vi "SMain.vi"() -> ()   [LabVIEW 2011] (continued)
                              tunnel: w1059 -> [_ w1085]
                              tunnel: w1058 -> [_ w1084]
                              tunnel: [TRUE ("Total Reult") w1083] -> w1057
                              tunnel: [_ w1082] -> w1056
                              tunnel: w1055 -> [_ w1081]
                              tunnel: w1054 -> [_ w1080]
                              tunnel: w1053 -> [_ w1079]
                              tunnel: w1052 -> [_ w1078]
                              tunnel: w1050 -> [_ w1077]
                              tunnel: [string[] [] ("NEXT Pair Name") w1076] -> w1047
                              tunnel: [bool[] [TRUE] ("Testing Results") w1075] -> w1046
                              frame False {
                              }
                              frame True {
                                n626 = stacked-sequence {
                                seq-local: [_ w1131] -> [_ _]
                                tunnel: w1095 -> [w1097 _]
                                tunnel: w1094 -> [w1098 _]
                                tunnel: w1093 -> [_ _]
                                tunnel: w1092 -> [_ _]
                                tunnel: w1091 -> [w1113 _]
                                tunnel: w1090 -> [_ w1137]
                                tunnel: w1089 -> [_ w1138]
                                tunnel: w1088 -> [w1105 _]
                                tunnel: w1087 -> [w1117 _]
                                tunnel: w1086 -> [w1104 _]
                                tunnel: w1085 -> [_ w1136]
                                tunnel: w1084 -> [w1101 _]
                                tunnel: [_ w1131] -> w1083
                                tunnel: [_ w1135] -> w1082
                                tunnel: w1081 -> [_ w1134]
                                tunnel: w1080 -> [_ w1133]
                                tunnel: w1079 -> [_ _]
                                tunnel: w1078 -> [_ _]
                                tunnel: w1077 -> [_ w1129]
                                tunnel: [_ w1127] -> w1076
                                tunnel: [_ w1126] -> w1075
                                frame #0 {
                                w1107 = "MDNEXT" ("元素")
                                w1119 = u16 0 items=["Normal Input", "Start", "Product Inf", "End"] ("Summary Method")
                                n627 = local read "Diff Test Item smooth"() -> (w1100:string[])
                                n628 = Build Array("NEXT" ("元素")) -> (w1108:string[])
                                n629 = local read "Length"() -> (w1102:string)
                                n630 = Search 1D Array(1D array=w1101, element=w1107) -> (index of element=w1111:i32)  [unwired: 1 in]
                                n631 = Not Equal?(x=w1111, y=-1) -> (x != y?=w1109:bool)
                                n632 = case shown="真" w1109 {
                                tunnel: w1108 -> [w1120 w1123]
                                tunnel: w1107 -> [_ w1122]
                                tunnel: [w1120 w1121] -> w1103
                                frame False {
                                }
                                frame True {
                                n633 = Build Array (concatenate)(w1123, w1122) -> (w1121:string[])
                                }
                                }
                                "NEXTList" <- w1103
                                n634 = local read "smooth point"() -> (w1099:i32)
                                n635 = call "Summary Generating.vi"("Summary Method"=w1119, "Status String"=w1117, "String 2"="NEXT Testing....." ("Test Status:")) -> ()  [unwired: 25 in]
                                n636 = local read "Switch array"() -> (w1114:bool[][])
                                n637 = local read "S-Pair Loop"() -> (w1115:i32)
                                n638 = Bundle("DAQ Device"=w1113, "Switch array"=w1114, "S-Pair Loop"=w1115) -> (w1112:T24)  [unwired: 1 in]
                                n639 = local write "Matrix In"(w1112) -> ()
                                n640 = Bundle By Name(cluster="Information In 2", "Sample PN:"=w1105, "SampleSN:"=w1104, "Sparam Test Item"=w1103, "S-para Pair Name"=w1097, "Length"=w1102, "Diff Test Item Name"=w1101, "Diff Test Item Name smooth"=w1100, "smooth point"=w1099, "limitSpec"=w1098) -> (→"NEXT INF":T4)
                                }
                                frame #1 {
                                n641 = local read "NEXT INF"() -> (w1124:T4)
                                n642 = local read "proBar_ref"() -> (w1128:refnum<vi>)
                                n643 = local read "Reference"() -> (w1125:T5)
                                n644 = local read "Matrix In"() -> (w1140:T13)
                                n645 = local read "Option"() -> (w1130:T11)
                                n646 = call "Sparameter Testing.vi"("VNA Model:"=w1138, "VNA VISA"=w1137, "Port Type"=w1136, "Reference"=w1125, "VISA COM"=w1134, "Information In"=w1124, "Mode(Demo,Manual)"=w1129, "DAQ  Model:"=w1133, "S4P Data Type"=enum16{"THRU", "NEXT", "FEXT"}."NEXT", "Matrix  In"=w1140, "Option"=w1130, "proBar_ref"=w1128) -> ("String data"=w1135:string, "Testing Results"=w1126:bool[], "Total Reult"=w1131:bool, "Items Result"=→"NEXT Result":string[])  [unwired: 6 in, 6 out]
                                n647 = Unbundle By Name(w1124) -> ("S-para Pair Name"=w1127:string[])
                                }
                                }
                              }
                            }
                            "NEXTReult" <- w1057
                            "NEXT String data" <- w1056
                            "NEXTList" <- w1047
                            "NEXTReults" <- w1046
                          }
                          frame #5 {
                            n648 = local read "Diff Test Item Name"() -> (w1152:string[])
                            n649 = local read "limitSpec"() -> (w1142:string[][])
                            n650 = local read "Urgent Stop"() -> (w1146:bool)
                            n651 = local read "FEXT Pair Name"() -> (w1153:string[])
                            n652 = Search 1D Array(1D array=w1152, element="FEXT" ("元素")) -> (index of element=w1162:i32)  [unwired: 1 in]
                            n653 = Bundle("Demo"=w1144, "Manual"=w1143, "Urgent Stop"=w1146) -> (w1145:T21)  [unwired: 1 in]
                            n654 = Not Equal?(x=w1162, y=-1) -> (x != y?=w1163:bool)
                            "FEXT?" <- w1163
                            n655 = case shown="真" w1163 {
                              tunnel: w1153 -> [_ w1186]
                              tunnel: w1142 -> [_ w1185]
                              tunnel: w1155 -> [_ w1184]
                              tunnel: w1162 -> [_ w1183]
                              tunnel: w1161 -> [_ w1182]
                              tunnel: w1160 -> [_ w1181]
                              tunnel: w1159 -> [_ w1180]
                              tunnel: w1158 -> [_ w1179]
                              tunnel: w1157 -> [_ w1178]
                              tunnel: w1144 -> [_ w1177]
                              tunnel: w1156 -> [_ w1176]
                              tunnel: w1154 -> [_ w1175]
                              tunnel: w1152 -> [_ w1174]
                              tunnel: [TRUE ("Total Reult") w1173] -> w1151
                              tunnel: [_ w1172] -> w1150
                              tunnel: w1149 -> [_ w1171]
                              tunnel: w1148 -> [_ w1170]
                              tunnel: w1147 -> [_ w1169]
                              tunnel: w1145 -> [_ w1168]
                              tunnel: [_ w1167] -> w1141
                              frame False {
                              }
                              frame True {
                                n656 = stacked-sequence {
                                seq-local: [_ w1222 _] -> [_ _ _]
                                tunnel: w1186 -> [w1193 _ _]
                                tunnel: w1185 -> [w1188 _ _]
                                tunnel: w1184 -> [_ _ _]
                                tunnel: w1183 -> [_ _ _]
                                tunnel: w1182 -> [w1207 _ _]
                                tunnel: w1181 -> [_ w1229 _]
                                tunnel: w1180 -> [_ w1230 _]
                                tunnel: w1179 -> [w1196 _ _]
                                tunnel: w1178 -> [w1210 _ _]
                                tunnel: w1177 -> [_ _ _]
                                tunnel: w1176 -> [w1195 _ _]
                                tunnel: w1175 -> [_ w1228 _]
                                tunnel: w1174 -> [w1191 _ _]
                                tunnel: [_ w1222 _] -> w1173
                                tunnel: [_ w1226 _] -> w1172
                                tunnel: w1171 -> [_ w1225 _]
                                tunnel: w1170 -> [_ w1224 _]
                                tunnel: w1169 -> [_ _ _]
                                tunnel: w1168 -> [_ w1220 _]
                                tunnel: [_ w1217 _] -> w1167
                                frame #0 {
                                w1198 = "MDFEXT" ("元素")
                                w1212 = u16 0 items=["Normal Input", "Start", "Product Inf", "End"] ("Summary Method")
                                n657 = local read "Diff Test Item smooth"() -> (w1190:string[])
                                n658 = local read "smooth point"() -> (w1189:i32)
                                n659 = Search 1D Array(1D array=w1191, element=w1198) -> (index of element=w1202:i32)  [unwired: 1 in]
                                n660 = Not Equal?(x=w1202, y=-1) -> (x != y?=w1200:bool)
                                n661 = Build Array("FEXT" ("元素")) -> (w1199:string[])
                                n662 = case shown="假" w1200 {
                                tunnel: w1199 -> [w1213 w1216]
                                tunnel: w1198 -> [_ w1215]
                                tunnel: [w1213 w1214] -> w1194
                                frame False {
                                }
                                frame True {
                                n663 = Build Array (concatenate)(w1216, w1215) -> (w1214:string[])
                                }
                                }
                                "FEXTLIst" <- w1194
                                n664 = call "Summary Generating.vi"("Summary Method"=w1212, "Status String"=w1210, "String 2"="FEXT Testing....." ("Test Status:")) -> ()  [unwired: 25 in]
                                n665 = local read "S-Pair Loop"() -> (w1204:i32)
                                n666 = local read "N-Pair Loop"() -> (w1205:i32)
                                n667 = local read "Switch array"() -> (w1208:bool[][])
                                n668 = local read "Length"() -> (w1192:string)
                                n669 = Add(x=w1204, y=w1205) -> (x+y=w1203:i32)
                                n670 = Bundle("DAQ Device"=w1207, "Switch array"=w1208, w1203) -> (w1206:T22)  [unwired: 1 in]
                                n671 = Bundle By Name(cluster=T4 {"Sample PN: "="", "SampleSN:"="", "Sparam Test Item"=[], "S-para Pair Name"=[], "Length"="", "Diff Test Item Name"=["SDD21", "SDD22", "SCD21", "SCD22", "SCC11", "NEXT", "FEXT"], "Diff Test Item Name smooth"=[], "smooth point"=0.0, "limitSpec"=[], "switchIndexOffset"=0, "testType"=enum."Loss", "pairStartIndex"=0, "DAQ  Model:"=enum."NI PCI-6509", "VISA COM"="", "Matrix  In"=[]} ("Information In 3"), "Sample PN:"=w1196, "SampleSN:"=w1195, "Sparam Test Item"=w1194, "S-para Pair Name"=w1193, "Length"=w1192, "Diff Test Item Name"=w1191, "Diff Test Item Name smooth"=w1190, "smooth point"=w1189, "limitSpec"=w1188) -> (→"FEXT INF":T4)
                                n672 = local write "Matrix In"(w1206) -> ()
                                }
                                frame #1 {
                                n673 = local read "FEXT INF"() -> (w1218:T4)
                                n674 = local read "Reference"() -> (w1227:T5)
                                n675 = local read "proBar_ref"() -> (w1219:refnum<vi>)
                                n676 = local read "Matrix In"() -> (w1232:T13)
                                n677 = local read "Option"() -> (w1221:T11)
                                n678 = call "Sparameter Testing.vi"("VNA Model:"=w1230, "VNA VISA"=w1229, "Port Type"=w1228, "Reference"=w1227, "VISA COM"=w1225, "Information In"=w1218, "Mode(Demo,Manual)"=w1220, "DAQ  Model:"=w1224, "S4P Data Type"=enum16{"THRU", "NEXT", "FEXT"}."FEXT", "Matrix  In"=w1232, "Option"=w1221, "proBar_ref"=w1219) -> ("String data"=w1226:string, "Testing Results"=w1217:bool[], "Total Reult"=w1222:bool, "Items Result"=→"FEXT Result":string[])  [unwired: 6 in, 6 out]
                                }
                                frame #2 {
                                }
                                }
                              }
                            }
                            "FEXTReult" <- w1151
                            "FEXT String data" <- w1150
                            "FEXT Results" <- w1141
                          }
                          frame #6 {
                            # "save general"
                            n679 = local read "VNA Model:"() -> (w1240:enum16{"E5071C", "N5230A(C)", "N5224A"})
                            n680 = property on="Approval:" class="Ring (严格)"() -> ("RingText.Text"=w1243:string)  [unwired: 2 in, 2 out]
                            n681 = property on="Tester:" class="Ring (严格)"() -> ("RingText.Text"=w1244:string)  [unwired: 2 in, 2 out]
                            n682 = local read "NEXTList"() -> (w1255:string[])
                            n683 = local read "SparaReults"() -> (w1252:bool[])
                            n684 = local read "itemList"() -> (w1256:string[])
                            n685 = local read "NEXTReults"() -> (w1251:bool[])
                            n686 = local read "FEXT Results"() -> (w1250:bool[])
                            n687 = local read "FEXTLIst"() -> (w1254:string[])
                            n688 = local read "Applicant:"() -> (w1247:string)
                            n689 = local read "PN Des"() -> (w1246:string)
                            n690 = local read "Report No."() -> (w1242:string)
                            n691 = local read "P/N:"() -> (w1245:string)
                            n692 = local read "Sample #"() -> (w1241:string)
                            n693 = Insert Into Array(array=w1252, new element #1=w1251, new element #2=w1250) -> (w1249:bool[])  [unwired: 1 in]
                            n694 = Insert Into Array(array=w1256, new element #1=w1255, new element #2=w1254) -> (w1253:string[])  [unwired: 1 in]
                            n695 = call "getReportMsg.vi"("partDescription"=w1246, "partNo"=w1245, "fixtureSerialNo"="Fixture No", "preparedBy"=w1244, "approvedBy"=w1243, "temprature"="Temperature(℃)", "VNA Model:"=w1240, "reportNo"=w1242, "application"=w1247, "sampleNo"=w1241, "rHumidity"="Relative Humidity(%)") -> ("value"=w1238:string[], "item"=w1239:string[])  [unwired: 7 in]
                            n696 = for {
                              tunnel: w1249 -> [w1260] mode=indexing
                              tunnel: [w1257] -> w1248 mode=indexing
                              n697 = Select(t="Pass", s=w1260, f="Fail") -> (s? t:f=w1257:string)
                            }
                            n698 = local read "TXT Data Path"() -> (w1234:path)
                            n699 = call "saveGeneral.vi"("itemList"=w1253, "resultsStr"=w1248, "item"=w1239, "文件（使用对话框）"=w1234, "value"=w1238) -> ("cluResult"=→"cluResult":T2)  [unwired: 6 in, 4 out]
                          }
                          frame #7 {
                            n700 = case shown="假" w1261 {
                              tunnel: [w1272 w1275] -> w1266
                              frame False {
                                n701 = local read "original Path"() -> (w1274:path)
                                n702 = Build Path(base path=w1274, name or relative path="TXT" ("名称或相对路径")) -> (appended path=w1272:path)
                              }
                              frame True {
                                n703 = call <vilib>:"Application Directory.vi"() -> ("Application Directory"=w1277:path)
                                n704 = Build Path(base path=w1277, name or relative path="Demo_data") -> (appended path=w1275:path)
                              }
                            }
                            n705 = local read "S-para Pair Name"() -> (w1267:string[])
                            n706 = local read "S-Para Item List"() -> (w1268:string[])
                            n707 = local read "frePoints"() -> (w1265:string[])
                            n708 = call "采集频点值.vi"("频率点（MHZ）"=w1265, "测试对名称"=w1267, "S参数测试项目"=w1268, "TXT文件所处路径"=w1266) -> ("测试项目及频点在DB输出"=w1263:string, "测试项目及频点在txt输出"=→"测试项目及频点在txt输出":string)
                            n709 = control-ref of="db_ResultString"() -> (w1271:refnum<vi>)
                            n710 = property class="Str"(reference=w1271) -> (reference out=w1262:refnum<vi>, "Value"=w1270:string)  [unwired: 1 in, 1 out]
                            n711 = Concatenate Strings(w1270, w1263) -> (w1269:string)
                            n712 = property class="Str"(reference=w1262, "Value"=w1269) -> ()  [unwired: 1 in, 2 out]
                          }
                          frame #8 {
                            # "烧录、检验EEPROM"
                            n713 = local read "EEPROMTF"() -> (w1280:bool)
                            n714 = local read "EE Write"() -> (w1279:bool)
                            n715 = And(x=w1280, y=w1279) -> (x .and. y?=w1278:bool)
                            n716 = case shown="真" w1278 {
                              tunnel: w1281 -> [w1286 w1312]
                              frame False {
                                n717 = property class="Str"(reference=w1286) -> (reference out=w1282:refnum<vi>, "Value"=w1285:string)  [unwired: 1 in, 1 out]
                                n718 = local write "EEResult"(TRUE ("EEResult")) -> ()
                                n719 = Concatenate Strings(w1285, "\nEEPROM write option not selected：EEPROM need not burn\n" ("字符串")) -> (w1284:string)
                                n720 = property class="Str"(reference=w1282, "Value"=w1284) -> ()  [unwired: 1 in, 2 out]
                              }
                              frame True {
                                w1291 = "\n"
                                n721 = local read "mid_str_labelType"() -> (w1309:string)
                                n722 = local read "PN description"() -> (w1289:string)
                                n723 = local read "RS232 I2C VISA"() -> (w1311:refnum<visa-resource-name>)
                                n724 = local read "mid_array_temp_int"() -> (w1304:u8[][])
                                n725 = local read "Adaptor:"() -> (w1310:enum16{"RS232 - IIC", "LUXSHARE - IIC"})
                                n726 = Concatenate Strings(w1309, w1289) -> (w1306:string)
                                n727 = property class="Str"(reference=w1312) -> (reference out=w1293:refnum<vi>, "Value"=w1300:string)  [unwired: 1 in, 1 out]
                                n728 = call "readLabelTypeForH3C.vi"("input_str_labelType"=w1306) -> ("show_str_011string"=w1288:string)  [unwired: 1 out]
                                n729 = flat-sequence {
                                tunnel: w1311 -> [w1316]
                                tunnel: w1310 -> [w1317]
                                tunnel: w1304 -> [w1319]
                                tunnel: w1288 -> [w1318]
                                tunnel: [w1317] -> w1308
                                tunnel: [w1316] -> w1307
                                tunnel: w1306 -> [w1315]
                                tunnel: [w1315] -> w1305
                                tunnel: w1304 -> [w1314]
                                tunnel: [w1314] -> w1303
                                tunnel: ["Write EEprom"] -> w1292
                                tunnel: w1308 -> [w1326]
                                tunnel: w1307 -> [w1325]
                                tunnel: w1305 -> [w1324]
                                tunnel: w1303 -> [w1322]
                                tunnel: [w1323] -> w1302
                                tunnel: [w1322] -> w1301
                                tunnel: [w1321] -> w1296
                                tunnel: ["Read EEprom"] -> w1290
                                tunnel: w1302 -> [w1329]
                                tunnel: w1301 -> [w1331]
                                tunnel: [w1330] -> w1299
                                tunnel: [w1329] -> w1298
                                tunnel: [w1328] -> w1297
                                tunnel: w1296 -> [w1327]
                                tunnel: [w1327] -> w1295
                                tunnel: w1298 -> [w1340]
                                tunnel: w1297 -> [w1338]
                                tunnel: w1295 -> [w1339]
                                tunnel: w1294 -> [w1341]
                                tunnel: w1293 -> [w1342]
                                frame #0 {
                                n730 = call "EEPROM烧录模块.vi"("input_array_temp_int"=w1319, "input_str_011string"=w1318, "Visa Port :"=w1316, "Adaptor:"=w1317) -> ()  [unwired: 6 in, 2 out]
                                }
                                frame #1 {
                                n731 = call "EEPROM读取模块.vi"("input_array_temp_int"=w1322, "input_str_labelType"=w1324, "VISA :"=w1325, "Adaptor"=w1326) -> ("pagesEqual00?"=w1321:bool, "show_array_read_int"=w1323:u8[][])  [unwired: 6 in]
                                }
                                frame #2 {
                                n732 = call "compareTempAndRead.vi"("input_array_temp"=w1331, "input_array_read"=w1329) -> ("show_str_message"=w1330:string, "show_testResult"=w1328:bool)  [unwired: 8 in]
                                }
                                frame #3 {
                                n733 = local read "original Path"() -> (w1335:path)
                                n734 = local read "Demo"() -> (w1336:bool)
                                n735 = And(x=w1339, y=w1338) -> (x .and. y?=→"EEResult":bool)
                                n736 = Build Path(base path=w1335, name or relative path="TXT" ("名称或相对路径")) -> (appended path=w1334:path)
                                n737 = Select(t=w1335, s=w1336, f=w1334) -> (s? t:f=w1333:path)
                                n738 = call "saveEEPFiles2.vi"("input_path"=w1333, "input_array_read_int"=w1340) -> ()  [unwired: 10 in]
                                }
                                frame #4 {
                                n739 = property class="Str"(reference=w1342, "Value"=w1341) -> ()  [unwired: 1 in, 2 out]
                                }
                                }
                                n740 = Concatenate Strings(w1300, w1291, w1292, w1291, w1290, w1291, w1299) -> (w1294:string)
                              }
                            }
                          }
                          frame #9 {
                            # "打印标签"
                            n741 = Not(x=w1343) -> (.not. x?=w1344:bool)
                            n742 = case shown="假" w1344 {
                              tunnel: w1345 -> [w1357 w1425]
                              frame True {
                                (unwired) "0. P/N  luxshare\n1. AWG\n2. Length（不可用）\n3. SN\n4. Custmer PN "  # Data In Format
                                n743 = local read "SparaReult"() -> (w1354:bool)
                                n744 = local read "NEXTReult"() -> (w1353:bool)
                                n745 = local read "FEXTReult"() -> (w1352:bool)
                                n746 = local read "EEResult"() -> (w1350:bool)
                                n747 = local read "LabelTF"() -> (w1351:bool)
                                n748 = local write "proBar"(u8 96 ("proBar")) -> ()
                                n749 = Compound Arithmetic op=AND(w1350, w1354, w1353, w1352, w1351) -> (w1348:bool)
                                n750 = property class="Str"(reference=w1357) -> (reference out=w1356:refnum<vi>, "Value"=w1355:string)  [unwired: 1 in, 1 out]
                                n751 = Or(x=w1348, y=FALSE) -> (x .or. y?=w1346:bool)
                                n752 = case shown="真" w1346 {
                                tunnel: w1356 -> [w1359 w1363]
                                tunnel: w1355 -> [w1361 w1364]
                                frame False {
                                n753 = Concatenate Strings(w1361, "\nNo Label has been printed!\n") -> (w1358:string)
                                n754 = property class="Str"(reference=w1359, "Value"=w1358) -> ()  [unwired: 1 in, 2 out]
                                n755 = local write "条码输出"("nolabel" ("条码输出")) -> ()
                                }
                                frame True {
                                n756 = stacked-sequence {
                                seq-local: [w1366 _ _ _] -> [_ w1377 _ _]
                                seq-local: [_ w1376 _ _] -> [_ _ w1401 _]
                                tunnel: w1364 -> [w1368 _ _ _]
                                tunnel: w1363 -> [w1365 w1374 w1402 _]
                                frame #0 {
                                n757 = Concatenate Strings(w1368, "\nLabel Printe Command Was Sent. \n") -> (w1366:string)
                                n758 = property class="Str"(reference=w1365, "Value"=w1366) -> ()  [unwired: 1 in, 2 out]
                                }
                                frame #1 {
                                n759 = vi-ref "打标签模式选择.vi"() -> (w1386:refnum<vi>)
                                n760 = property class="VI"(reference=w1386) -> ("Name"=w1385:string)  [unwired: 1 in, 2 out]
                                n761 = local read "midVar_time_date"() -> (w1394:timestamp)
                                n762 = local read "midVar_str_SN"() -> (w1395:string)
                                n763 = local read "Printer VISA"() -> (w1391:refnum<visa-resource-name>)
                                n764 = local read "Label Type"() -> (w1393:string[])
                                n765 = local read "LabelNum"() -> (w1390:i32)
                                n766 = local read "Data In"() -> (w1392:string[])
                                n767 = Open VI Reference(type specifier VI Refnum (for type only)=refnum<vi> refnum ("类型说明符VI引用句柄（仅用于类型）"), vi path=w1385, options=128 ("选项")) -> (vi reference=w1382:refnum<vi>, error out=w1378:errorcluster)  [unwired: 3 in]
                                n768 = local read "打印模式"() -> (w1389:enum16{"IT Print", "EE Print"})
                                n769 = local read "PRINT"() -> (w1387:refnum<k24>)
                                n770 = local read "SN"() -> (w1388:refnum<k24>)
                                n771 = call-by-ref "Start Asynchronous Call"(reference=w1382, error in=w1378, "LabelNum"=w1390, "Printer VISA"=w1391, "Data In"=w1392, "Label Type"=w1393, "midVar_time_date"=w1394, "打印模式"=w1389, "midVar_str_SN"=w1395, "引用"=w1388, "print path local"="Fast Print", "PRINT"=w1387, "错误输入（无错误）"="错误输入（无错误）", "条码类型"="制程条码") -> (reference out=w1380:refnum<vi>, error out=w1373:errorcluster)  [unwired: 4 in, 4 out]
                                n772 = flat-sequence {
                                tunnel: w1380 -> [w1396]
                                tunnel: [w1396] -> w1379
                                frame #0 {
                                n773 = Wait (ms)(milliseconds to wait=u32 1500 ("等待时间（毫秒）")) -> ()  [unwired: 1 out]
                                }
                                }
                                n774 = Unbundle(w1373) -> ("source"=w1372:string)  [unwired: 2 out]
                                n775 = local write "labelFlag"(TRUE ("labelFlag")) -> ()
                                n776 = Concatenate Strings(w1377, w1372, "\n") -> (w1376:string)
                                n777 = Close Reference(reference=w1379) -> ()  [unwired: 1 in, 1 out]
                                n778 = property class="Str"(reference=w1374, "Value"=w1376) -> ()  [unwired: 1 in, 2 out]
                                }
                                frame #2 {
                                n779 = local read "S/N:"() -> (w1400:string)
                                n780 = Concatenate Strings(w1400, " :Test Finished !" ("字符串")) -> (w1398:string)
                                n781 = Concatenate Strings(w1401, "\nLabel has been printed!\n", w1398) -> (w1403:string)
                                n782 = property class="Str"(reference=w1402, "Value"=w1403) -> ()  [unwired: 1 in, 2 out]
                                }
                                frame #3 {
                                n783 = local read "P/N:"() -> (w1412:string)
                                n784 = local read "Impedance Spec String"() -> (w1407:string)
                                n785 = local read "Current Testing Label/当前测试条码"() -> (w1411:string)
                                n786 = local read "original Path"() -> (w1410:path)
                                n787 = Build Path(base path=w1410, name or relative path="TXT" ("名称或相对路径")) -> (appended path=w1408:path)
                                n788 = call "TDD一致性检查.vi"("TDD filePath"=w1408, "Spec String"=w1407, "SN"=w1411, "PN"=w1412) -> ("报警颜色"=w1405:string, "判定"=w1406:bool)  [unwired: 6 in]
                                n789 = case shown="假" w1406 {
                                tunnel: w1405 -> [w1414 _]
                                frame False {
                                n790 = control-ref of="Test Status:"() -> (w1415:refnum<vi>)
                                n791 = call "颜色常量（汉字）.vi"("颜色"=w1414) -> ("颜色常量"=w1413:u32)  [unwired: 10 in]
                                n792 = property on="属性节点" class="Str"(reference=w1415, "Text.BGColor"=w1413, "Text.TextColor"=u32 0) -> ()  [unwired: 1 in, 2 out]
                                }
                                frame True {
                                }
                                }
                                }
                                }
                                }
                                }
                              }
                              frame False {
                                (unwired) "0. P/N  luxshare\n1. AWG\n2. Length（不可用）\n3. SN\n4. Custmer PN "  # Data In Format
                                n793 = local write "proBar"(u8 96 ("proBar")) -> ()
                                n794 = property class="Str"(reference=w1425) -> (reference out=w1421:refnum<vi>, "Value"=w1424:string)  [unwired: 1 in, 1 out]
                                n795 = local read "S/N:"() -> (w1419:string)
                                n796 = disable-structure shown="禁用" {
                                frame Disabled {
                                n797 = local read "midVar_time_date"() -> (w1434:timestamp)
                                n798 = local read "midVar_str_SN"() -> (w1433:string)
                                n799 = local read "Printer VISA"() -> (w1429:refnum<visa-resource-name>)
                                n800 = local read "Label Type"() -> (w1435:string[])
                                n801 = local read "LabelNum"() -> (w1437:i32)
                                n802 = local read "Data In"() -> (w1436:string[])
                                n803 = local read "PRINT"() -> (w1427:refnum<k24>)
                                n804 = local read "SN"() -> (w1426:refnum<k24>)
                                n805 = local read "打印模式"() -> (w1432:enum16{"IT Print", "EE Print"})
                                n806 = call "打标签模式选择.vi"("LabelNum"=w1437, "Printer VISA"=w1429, "Data In"=w1436, "Label Type"=w1435, "midVar_time_date"=w1434, "打印模式"=w1432, "midVar_str_SN"=w1433, "引用"=w1426, "print path local"=TRUE, "PRINT"=w1427) -> ("labelFlag"=w1431:bool, "条码输出"=w1430:string)  [unwired: 6 in, 2 out]
                                n807 = local write "labelFlag"(w1431) -> ()
                                n808 = local write "条码输出"(w1430) -> ()
                                }
                                frame Enabled {
                                }
                                }
                                n809 = Concatenate Strings(w1419, " :Test Finished !" ("字符串")) -> (w1417:string)
                                n810 = Concatenate Strings(w1424, "\nDemo mode Label has been printed!\n", w1417) -> (w1420:string)
                                n811 = property class="Str"(reference=w1421, "Value"=w1420) -> ()  [unwired: 1 in, 2 out]
                              }
                            }
                          }
                          frame #10 {
                            n812 = property class="Str"(reference=w1441) -> ("Value"=w1440:string)  [unwired: 1 in, 2 out]
                            n813 = local read "测试项目及频点在txt输出"() -> (w1438:string)
                            n814 = Concatenate Strings(w1440, w1438) -> (w1439:string)
                          }
                          frame #11 {
                            w1482 = u16 3 items=["Normal Input", "Start", "Product Inf", "End"] ("Summary Method")
                            n815 = Or(x=w1477, y=w1476) -> (x .or. y?=w1475:bool)
                            n816 = local write "proBar"(u8 97 ("proBar")) -> ()
                            n817 = case shown="假" w1475 {
                              tunnel: w1483 -> [w1487 _]
                              tunnel: w1473 -> [w1486 _]
                              tunnel: w1474 -> [w1485 _]
                              tunnel: [w1484 "demo or manual mode" ("source")] -> w1442
                              frame False {
                                n818 = case shown="\"LX MCU\"" w1486 {
                                tunnel: w1487 -> [w1492 _ _]
                                tunnel: w1485 -> [_ w1496 w1500]
                                tunnel: [w1488 w1493 w1498] -> w1484
                                frame "NI PCI-6509", Default {
                                n819 = local read "Switch array"() -> (w1490:bool[][])
                                n820 = call "6509 simple.vi"("index (row)"=i8 79, "array input: P0-P1-P2-P3-P4-P5"=w1490, "DAQ device"=w1492) -> ("error out"=w1489:errorcluster)  [unwired: 4 in]
                                n821 = Unbundle By Name(w1489) -> ("source"=w1488:string)  [unwired: 2 out]
                                }
                                frame "LX MCU" {
                                w1495 = u16 1 items=["Testing", "Close All"] ("Function")
                                n822 = call "MCU Switch Control.vi"("Function"=w1495, "VISA"=w1496) -> ("error out"=w1494:errorcluster)  [unwired: 9 in]
                                n823 = Unbundle By Name(w1494) -> ("source"=w1493:string)  [unwired: 2 out]
                                }
                                frame "LX MCU_40G" {
                                w1499 = u16 1 items=["Testing", "Close All"] ("Function")
                                n824 = call "40G MCU Switch Control.vi"("Function"=w1499, "VISA"=w1500) -> ("error out"=w1497:errorcluster)  [unwired: 9 in]
                                n825 = Unbundle By Name(w1497) -> ("source"=w1498:string)  [unwired: 2 out]
                                }
                                }
                              }
                              frame True {
                              }
                            }
                            n826 = local read "Start Time"() -> (w1479:timestamp)
                            n827 = Get Date/Time In Seconds() -> (seconds since 1Jan1904=w1478:timestamp)
                            n828 = Subtract(x=w1478, y=w1479) -> (x-y=w1480:dbl)
                            n829 = Number To Fractional String(number=w1480) -> (F-format string=w1465:string)  [unwired: 3 in]
                            n830 = call "Summary Generating.vi"("Summary Method"=w1482, "Status String"=w1481, "Test Taking Time(s)"=w1465) -> ()  [unwired: 25 in]
                            n831 = Concatenate Strings("switch status:" ("字符串"), w1442) -> (w1461:string)
                            n832 = local read "SparaReult"() -> (w1459:bool)
                            n833 = local read "NEXTReult"() -> (w1458:bool)
                            n834 = local read "FEXTReult"() -> (w1457:bool)
                            n835 = local read "EEResult"() -> (w1449:bool)
                            n836 = Compound Arithmetic op=AND(w1459, w1458, w1457, w1449) -> (w1456:bool)
                            "test result" <- w1456
                            n837 = case shown="假" w1456 {
                              tunnel: [TRUE ("可见") TRUE ("可见")] -> w1455
                              tunnel: ["Testing Pass" ("文本.文本") "Testing Fail" ("文本.文本")] -> w1454
                              tunnel: [u32 6618880 u32 16711680] -> w1453
                              tunnel: [u32 40 ("文本.字体:字号") u32 40 ("文本.字体:字号")] -> w1452
                              frame True {
                              }
                              frame False {
                              }
                            }
                            n838 = property on="Result" class="Str"("Visible"=w1455, "Text.Text"=w1454, "Text.TextColor"=w1453, "Text.FontSize"=w1452, "DisabledEnum"=1, "Blinking"=FALSE ("闪烁")) -> ()  [unwired: 2 in, 2 out]
                            n839 = Format Date/Time String(time format string (%c)="%a %p %H:%M:%S %Y/%m/%d China Time.  Test Time: ") -> (date/time string=w1467:string)  [unwired: 2 in]
                            n840 = Format Date/Time String(time format string (%c)="%Y/%m/%d %H:%M:%S" ("时间格式字符串(%c)")) -> (date/time string=w1448:string)  [unwired: 2 in]
                            n841 = local read "test time"() -> (w1446:string[])
                            n842 = Concatenate Strings("Ended Test At " ("字符串"), w1467, w1465, "s" ("字符串"), "\n", w1461) -> (w1470:string)
                            n843 = call <vilib>:"Trim Whitespace.vi"("string"=w1448) -> ("trimmed string"=w1445:string)  [unwired: 1 in]
                            n844 = Concatenate Strings(w1464, "\r", w1470) -> (→"txt summary":string)
                            n845 = case shown="真" "Auto Count:" {
                              frame False {
                              }
                              frame True {
                                n846 = local read "Report No."() -> (w1514:string)
                                n847 = local read "Sample #"() -> (w1513:string)
                                n848 = local read "S/N:"() -> (w1515:string)
                                n849 = call "SN Report Number Increase.vi"("Sample #"=w1513, "Report No."=w1514, "S/N:"=w1515) -> ("Sample # out"=w1510:string, "Report No. out"=w1511:string, "S/N_out"=w1512:string)  [unwired: 6 in]
                                n850 = local write "S/N:"(w1512) -> ()
                                n851 = local write "Report No."(w1511) -> ()
                                n852 = local write "Sample #"(w1510) -> ()
                              }
                            }
                            n853 = Insert Into Array(array=w1446, new element=w1445) -> (w1444:string[])  [unwired: 1 in]
                            n854 = local write "test time"(w1444) -> ()
                          }
                          frame #12 {
                            n855 = local read "SparaReult"() -> (w1536:bool)
                            n856 = local read "NEXTReult"() -> (w1535:bool)
                            n857 = local read "FEXTReult"() -> (w1534:bool)
                            n858 = local read "EEResult"() -> (w1533:bool)
                            n859 = local read "SparaReults"() -> (w1525:bool[])
                            n860 = local read "NEXTReults"() -> (w1526:bool[])
                            n861 = property on="Test Status:" class="Str"() -> ("Value"=→"Test Status: 2":string)  [unwired: 2 in, 2 out]
                            n862 = Compound Arithmetic op=AND(w1536, w1535, w1534, w1533) -> (w1530:bool)
                            n863 = Insert Into Array(array=w1525, new element=w1526) -> (→"TestResult":bool[])  [unwired: 1 in]
                            n864 = local read "FullXml"() -> (w1518:bool)
                            n865 = local read "正常工单?"() -> (w1520:bool)
                            n866 = local read "打印模式"() -> (w1529:enum16{"IT Print", "EE Print"})
                            n867 = local read "测试模式"() -> (w1523:u16)
                            n868 = Equal?(x=w1523, y=u16 0) -> (x = y?=w1521:bool)
                            "测试模式" <- w1521
                            n869 = local read "EEUPLOAD"() -> (w1516:bool)
                            n870 = Equal?(x=w1529, y=enum16{"IT Print", "EE Print"}."IT Print") -> (x = y?=w1522:bool)
                            n871 = Compound Arithmetic op=AND(w1518, w1522, w1521, w1520) -> (w1517:bool)
                            n872 = Or(x=w1516, y=w1517) -> (x .or. y?=w1519:bool)
                            n873 = case shown="真" w1519 {
                              tunnel: w1531 -> [_ w1538]
                              tunnel: w1530 -> [_ w1537]
                              frame False {
                              }
                              frame True {
                                n874 = stacked-sequence {
                                seq-local: [w1554 _ _ _ _ _] -> [_ _ _ _ _ _]
                                seq-local: [w1553 _ _ _ _ _] -> [_ _ _ _ _ _]
                                tunnel: w1538 -> [_ _ _ _ _ _]
                                tunnel: w1537 -> [_ _ _ _ w1625 _]
                                frame #0 {
                                # "得到测试结果"
                                n875 = local read "条码输出"() -> (w1543:string)
                                n876 = property on="Current Testing Label/当前测试条码" class="Str"() -> ("Value"=w1552:string)  [unwired: 2 in, 2 out]
                                n877 = Equal?(x=w1543, y="nolabel") -> (x = y?=w1540:bool)
                                n878 = local read "Impedance Spec String"() -> (w1558:string)
                                n879 = String Length(string=w1543) -> (length=w1551:i32)
                                n880 = String Length(string=w1552) -> (length=w1550:i32)
                                n881 = local read "original Path"() -> (w1569:path)
                                n882 = local read "Diff Test Item Name"() -> (w1545:string[])
                                n883 = local read "TDR Test Item Name"() -> (w1544:string[])
                                n884 = call "_wmg_ImpSpecDivided@_XML.vi"("Input"=w1558, "input_dbl_stopTime"=2.0) -> ("OUTPUT2"=w1556:string[][], "Output"=w1557:string[][])
                                n885 = Greater?(x=w1550, y=w1551) -> (0:w1541:bool)
                                n886 = Or(x=w1541, y=w1540) -> (x .or. y?=w1539:bool)
                                n887 = Select(t=w1552, s=w1539, f=w1543) -> (s? t:f=→"usedSN":string)
                                n888 = Index Array(array=w1557, index (col) #1=0 ("禁用的索引 (列)"), index (col) #2=1 ("索引 (列)")) -> (element #1=w1585:string[], element #2=w1584:string[])  [unwired: 2 in]
                                n889 = Index Array(array=w1556, index (col)=1 ("禁用的索引 (列)")) -> (element=w1581:string[])  [unwired: 1 in]
                                n890 = Index Array(array=w1556, index (col)=3 ("禁用的索引 (列)")) -> (element=w1580:string[])  [unwired: 1 in]
                                n891 = Insert Into Array(array=w1545, new element=w1544) -> ()  [unwired: 1 in, 1 out]
                                n892 = call "readFromTXTForXMLFiles.vi"("input_path_dataSource"=w1569, "input_array_startTime"=w1585, "input_array_endTime"=w1584) -> ("show_Terminal Point"=w1554:dbl[], "show_array_TDD11"=→"show_TDD11":string[], "show_array_SDD21"=→"show_SDD21":string[], "show_array_SDD11_Max"=→"show_SDD11":string[], "show_array_ILD_Max"=→"show_ILD":string[], "show_array_SCC11_Max"=→"show_SCC11":string[], "show_array_Next"=→"show_Next":string[], "show_Cable Point"=w1553:dbl[], "show_array_TDD22"=→"show_TDD22":string[])  [unwired: 2 in, 2 out]
                                "show_Terminal Point" <- w1554
                                "show_Cable Point" <- w1553
                                n893 = Index Array(array=w1581, index #1=0 ("索引"), index #2=1 ("索引")) -> (element #1=w1573:string, element #2=w1570:string)
                                n894 = Index Array(array=w1580, index #1=0 ("索引"), index #2=1 ("索引")) -> (element #1=w1575:string, element #2=w1571:string)
                                n895 = local read "SparaReults"() -> (w1548:bool[])
                                n896 = local read "NEXTReults"() -> (w1547:bool[])
                                n897 = Insert Into Array(array=w1548, new element=w1547) -> (→"secondresult":bool[])  [unwired: 1 in]
                                n898 = Concatenate Strings(w1575, ":", w1573) -> (w1568:string)
                                n899 = Concatenate Strings(w1571, ":", w1570) -> (w1567:string)
                                n900 = Build Array(w1568, w1567) -> (→"show_impspec":string[])
                                }
                                frame #1 {
                                n901 = local read "TestResultSave"() -> (w1588:bool)
                                n902 = case shown="真" w1588 {
                                frame False {
                                }
                                frame True {
                                n903 = local read "auto get refer point"() -> (w1603:bool)
                                n904 = local read "width1"() -> (w1602:i32)
                                n905 = local read "width2"() -> (w1601:i32)
                                n906 = local read "show_TDD11"() -> (w1600:string[])
                                n907 = local read "show_TDD22"() -> (w1599:string[])
                                n908 = local read "test time"() -> (w1598:string[])
                                n909 = local read "show_impspec"() -> (w1597:string[])
                                n910 = local read "TestResult"() -> (w1589:bool[])
                                n911 = local read "FileName"() -> (w1596:string)
                                n912 = local read "FileVersion"() -> (w1595:string)
                                n913 = Bundle By Name(cluster="TestResultSummary", "auto get refer point"=w1603, "width1"=w1602, "width2"=w1601, "show_TDD11"=w1600, "show_TDD22"=w1599, "test time"=w1598, "show_impspec"=w1597, "TestResult"=w1589, "FileName"=w1596, "FileVersion"=w1595) -> (w1593:T9)
                                n914 = local read "original Path"() -> (w1592:path)
                                n915 = Build Path(base path=w1592, name or relative path="TXT\\TestResultSummary.txt" ("名称或相对路径")) -> (appended path=w1590:path)
                                n916 = call "TestResultSave.vi"("TestResultSummary"=w1593, "FileSavePath"=w1590) -> ()  [unwired: 10 in]
                                }
                                }
                                }
                                frame #2 {
                                n917 = local read "FileVersion"() -> (w1615:string)
                                n918 = local read "FileName"() -> (w1614:string)
                                n919 = local read "test time"() -> (w1619:string[])
                                n920 = local read "original Path"() -> (w1613:path)
                                n921 = local read "show_impspec"() -> (w1620:string[])
                                n922 = local read "usedSN"() -> (w1605:string)
                                n923 = local read "show_Terminal Point"() -> (w1618:dbl[])
                                n924 = local read "show_Cable Point"() -> (w1617:dbl[])
                                n925 = local read "sSpec"() -> (w1616:T3[])
                                n926 = local read "cluResult"() -> (w1612:T2)
                                n927 = Bundle By Name(cluster=T18 {"FileVersion"="DevelopmentSystem", "FileName"="DevelopmentSystem", "test time"=["2016/11/14 11:59:03"], "original Path"=path "D:/高频房软件/2. HPTS_VNA_Rev2.7.1.3-1107最新源码/Demo_data", "show_impspec"=[], "usedSN"="", "show_Terminal Point"=[], "show_Cable Point"=[], "sSpec"=[], "resultCluster"={"itemResult"=[], "itemName"=[]}, "customerPN"=""} ("xml_info"), "FileVersion"=w1615, "FileName"=w1614, "test time"=w1619, "original Path"=w1613, "show_impspec"=w1620, "usedSN"=w1605, "show_Terminal Point"=w1618, "show_Cable Point"=w1617, "sSpec"=w1616, "resultCluster"=w1612) -> (w1609:T18)
                                n928 = local read "TXT Data Path"() -> (w1611:path)
                                n929 = control-ref of="Test Status:"() -> (w1604:refnum<vi>)
                                n930 = local read "uploadPara"() -> (w1608:T1)
                                n931 = Build Path(base path=w1611, name or relative path="xml_info_new.txt") -> (appended path=w1606:path)
                                n932 = call "cluster_save.vi"("INI Fomatted Cluster"=w1609, "FileSavePath"=w1606) -> ()  [unwired: 9 in, 1 out]
                                n933 = local read "PN TYpe"() -> (w1607:string)
                                n934 = call "generateUploadZip.vi"("textRef"=w1604, "xmlPath"=w1606, "uploadPara"=w1608, "SN"=w1605, "pnType"=w1607) -> ()  [unwired: 14 in, 1 out]
                                }
                                frame #3 {
                                n935 = First Call?() -> (First Call?: T/F=w1622:bool)
                                n936 = case shown="真" w1622 {
                                frame False {
                                }
                                frame True {
                                (unwired) "net use \\\\172.20.20.86 Luxshare-ict /user:C040345" ("standard input")
                                n937 = local read "NetCmd"() -> (w1623:string)
                                n938 = call <vilib>:"System Exec.vi"("command line"=w1623) -> ()  [unwired: 7 in, 4 out]
                                }
                                }
                                }
                                frame #4 {
                                n939 = local read "CountXmlPath"() -> (w1626:path)
                                n940 = local read "usedSN"() -> (w1624:string)
                                n941 = call "xmlNodecreate.vi"("SN"=w1624, "TestResult"=w1625, "path"=w1626) -> ()  [unwired: 1 in, 1 out]
                                }
                                frame #5 {
                                n942 = local read "CountXmlPath"() -> (w1631:path)
                                n943 = call "xmlConfigRead.vi"("path to XML document"=w1631, "XPath expression"="//FailedSN/*") -> ("OutParaArray"=w1633:string[])  [unwired: 2 out]
                                n944 = call "xmlConfigRead.vi"("path to XML document"=w1631, "XPath expression"="//PassedSN/*") -> ("OutParaArray"=w1634:string[])  [unwired: 2 out]
                                n945 = Array Size(array=w1634) -> (size(s)=w1630:i32)
                                n946 = Array Size(array=w1633) -> (size(s)=w1629:i32)
                                n947 = Add(x=w1629, y=w1630) -> (x+y=w1628:i32)
                                n948 = Equal To 0?(x=w1628) -> (x = 0?=w1632:bool)
                                n949 = case shown="假" w1632 {
                                tunnel: w1629 -> [w1641 _]
                                tunnel: w1628 -> [w1639 _]
                                tunnel: [w1640 0.0] -> w1627
                                frame False {
                                n950 = Divide(x=w1641, y=w1639) -> (x/y=w1637:dbl)
                                n951 = Multiply(x=w1637, y=100) -> (x*y=w1640:dbl)
                                }
                                frame True {
                                }
                                }
                                n952 = local write "Passed"(w1630) -> ()
                                n953 = local write "Failed"(w1629) -> ()
                                n954 = local write "Total"(w1628) -> ()
                                n955 = local write "ratio"(w1627) -> ()
                                }
                                }
                              }
                            }
                          }
                          frame #13 {
                            n956 = property on="Tester:" class="Ring (严格)"() -> ("RingText.Text"=w1661:string)  [unwired: 2 in, 2 out]
                            n957 = property on="Approval:" class="Ring (严格)"() -> ("RingText.Text"=w1660:string)  [unwired: 2 in, 2 out]
                            n958 = local read "PN Des"() -> (w1665:string)
                            n959 = local read "P/N:"() -> (w1664:string)
                            n960 = Format Date/Time String(time format string (%c)="%Y-%m-%d") -> (date/time string=w1659:string)  [unwired: 2 in]
                            n961 = Build Array("Applicant:", w1665, w1664, "Report No.", "Sample #", w1661, w1660, w1659) -> (w1655:string[])
                            n962 = local read "Items Result"() -> (w1654:string[])
                            n963 = local read "EEResult"() -> (w1649:bool)
                            n964 = local read "FEXT Result"() -> (w1651:string[])
                            n965 = local read "NEXT Result"() -> (w1652:string[])
                            n966 = local read "NEXT?"() -> (w1657:bool)
                            n967 = local read "FEXT?"() -> (w1656:bool)
                            n968 = local read "Thru?"() -> (w1658:bool)
                            n969 = stacked-sequence {
                              frame #0 {
                                w1679 = ";" ("字符串")
                                n970 = local read "Reference"() -> (w1685:T5)
                                n971 = local read "SparaReult"() -> (w1672:bool)
                                n972 = local read "NEXTReult"() -> (w1671:bool)
                                n973 = local read "FEXTReult"() -> (w1670:bool)
                                n974 = local read "EEResult"() -> (w1669:bool)
                                n975 = Unbundle(w1685) -> ("db_ResultString"=w1684:refnum<vi>)  [unwired: 3 out]
                                n976 = property class="Str"(reference=w1684) -> ("Value"=w1677:string)  [unwired: 1 in, 2 out]
                                n977 = Compound Arithmetic op=AND(w1672, w1671, w1670, w1669) -> (w1668:bool)
                                n978 = local read "db_VNA"() -> (w1683:string)
                                n979 = Search and Replace String(replace all?=TRUE ("替换全部？(F)"), input string=w1677, search string="\n", replace string="," ("替换字符串(\"\")")) -> (result string=w1673:string)  [unwired: 4 in, 3 out]
                                n980 = Select(t="PASS", s=w1668, f="FAIL") -> (s? t:f=w1680:string)
                                n981 = Concatenate Strings(w1683, w1673, w1679, w1680, w1679) -> (w1678:string)
                                n982 = local write "db_VNA"(w1678) -> ()
                              }
                              frame #1 {
                                w1687 = ";" ("字符串")
                                n983 = local read "Applicant:"() -> (w1690:string)
                                n984 = local read "db_VNA"() -> (w1691:string)
                                n985 = property on="Tester:" class="Ring (严格)"() -> ("RingText.Text"=w1689:string)  [unwired: 2 in, 2 out]
                                n986 = property on="Approval:" class="Ring (严格)"() -> ("RingText.Text"=w1688:string)  [unwired: 2 in, 2 out]
                                n987 = Concatenate Strings(w1691, w1690, w1687, w1689, w1687, w1688, w1687) -> (w1686:string)
                                n988 = local write "db_VNA"(w1686) -> ()
                              }
                              frame #2 {
                                w1696 = ";" ("字符串")
                                n989 = local read "start"() -> (w1699:timestamp)
                                n990 = Get Date/Time In Seconds() -> (seconds since 1Jan1904=w1698:timestamp)
                                n991 = Subtract(x=w1698, y=w1699) -> (x-y=w1700:dbl)
                                n992 = Number To Fractional String(number=w1700, precision (6)=i16 2 ("精度(6)")) -> (F-format string=w1694:string)  [unwired: 2 in]
                                n993 = local read "db_VNA"() -> (w1705:string)
                                n994 = String To IP() -> (0:w1702:u32)  [unwired: 1 in]
                                n995 = Format Date/Time String(time format string (%c)="%H:%M:%S %Y/%m/%d") -> (date/time string=w1704:string)  [unwired: 2 in]
                                n996 = IP To String(2:w1702) -> (0:w1701:string)  [unwired: 1 in]
                                n997 = Concatenate Strings(w1694, "S" ("字符串")) -> (w1692:string)
                                n998 = Concatenate Strings(w1705, w1704, w1696, w1692, w1696, w1701, w1696, "EEPROM:OK", w1696) -> (w1703:string)
                                n999 = local write "db_VNA"(w1703) -> ()
                              }
                            }
                            n1000 = Build Array(w1658, w1657, w1656, w1649) -> (w1650:bool[])
                            n1001 = Build Array(w1654, w1652, w1651) -> (w1653:string[][])
                            n1002 = for {
                              tunnel: w1650 -> [w1710] mode=indexing
                              shift-right: [w1708] -> w1646
                              shift-left: w1655 -> [w1709]
                              tunnel: w1653 -> [w1707] mode=indexing
                              n1003 = case shown="真" w1710 {
                                tunnel: w1709 -> [w1711 w1716]
                                tunnel: [w1711 w1715] -> w1708
                                tunnel: w1707 -> [_ w1714]
                                frame False {
                                }
                                frame True {
                                n1004 = Array To Spreadsheet String(array=w1714, 3:"%s" ("格式字符串")) -> (spreadsheet string=w1713:string)  [unwired: 1 in]
                                n1005 = call <vilib>:"Trim Whitespace.vi"("string"=w1713) -> ("trimmed string"=w1712:string)  [unwired: 1 in]
                                n1006 = Insert Into Array(array=w1716, new element=w1712) -> (w1715:string[])  [unwired: 1 in]
                                }
                              }
                            }
                            "Report Inf" <- w1646
                            n1007 = local read "original Path"() -> (w1648:path)
                            n1008 = Array To Spreadsheet String(array=w1646, 3:"%s" ("格式字符串")) -> (spreadsheet string=w1645:string)  [unwired: 1 in]